vi "Remove signal offset - Intensity graph.vi"(8 "Y Scale.Offset and Multiplier":T2={"Offset"=-1.0, "Multiplier"=0.01}, 9 "X min & max":cluster{"X min":dbl, "X max":dbl}={"X min"=-0.4389, "X max"=0.4337}, 10 "Current offset to Subtract":T1, 11 "Data":dbl[][](graph)=array608x201[122208 elements]) -> (2 "element":dbl format="%#_6p", 3 "Data 2":dbl[][](graph))   [LabVIEW 2016]
uses:
  <vilib>/Utility/miscctls.llb/LVOffsetAndMultiplierTypeDef.ctl
panel:
  out "size(s)":i32[](array[numeric])=[608, 201]
  in  "Name":cluster{"X":string, "Y":string, "Z":string}={"X"="Vsd (V)", "Y"="VsgL (V)", "Z"="I (A)"}
  in  "Multiplier for Z":dbl=1.0
  out "Extracted offset signal":dbl[](graph)=[1.6161257772866977e-10, 1.6290791942826465e-10, 1.5574505344604935e-10, 1.336906684909418e-10, 1.3645714177751155e-10, 1.332223358181467e-10, 1.3050666232859227e-10, 1.2958403711911122e-10, 1.255087742878435e-10, 1.3438431801111367e-10, 1.3343613425025554e-10, 1.3796967145370057e-10, 1.3165183194433646e-10, 1.3668925850359432e-10, 1.3024287630588326e-10, 1.312700831203163e-10, 1.3321104247858227e-10, 1.3078678060118375e-10, 1.3530497739422364e-10, 1.3467471828812237e-10, 1.3723878465253679e-10, 1.3090930009882394e-10, 1.3122556497154024e-10, 1.3637331559158535e-10, 1.344618428788294e-10, 1.329384379410261e-10, 1.32436021964744e-10, 1.3267536092655857e-10, 1.3166939739249612e-10, 1.3315326666398787e-10, 1.3353313321086935e-10, 1.308474998524559e-10, 1.3430606449651886e-10, 1.3299895953833615e-10, 1.3379868824903194e-10, 1.3910099477931292e-10, 1.3013451141656342e-10, 1.3022082409430547e-10, 1.3957589625922564e-10, 1.353665592030564e-10, 1.3333443920084868e-10, 1.2848465625085147e-10, 1.3235016346451685e-10, 1.3493515356938516e-10, 1.3174423441498757e-10, 1.315524302167768e-10, 1.285457690751685e-10, 1.3328905759556557e-10, 1.3343261772296814e-10, 1.294368748288793e-10, 1.3434974891423252e-10, 1.2493174353418366e-10, 1.2818569417874195e-10, 1.375972145178948e-10, 1.3316519661996614e-10, 1.333160552162926e-10, 1.2807061594750737e-10, 1.2837747878228045e-10, 1.2925343445455244e-10, 1.3187529753832618e-10, 1.303560901885644e-10, 1.2711863941612015e-10, 1.2862070842066765e-10, 1.3111395651860157e-10, 1.2731619492783272e-10, 1.2928610264790122e-10, 1.3261741388716716e-10, 1.2936618128288814e-10, 1.3073484114123304e-10, 1.357022259458576e-10, 1.3308722303545194e-10, 1.2582991169744356e-10, 1.272984956323385e-10, 1.3313625085863706e-10, 1.3666798901102487e-10, 1.348284928206016e-10, 1.3155661735756067e-10, 1.2828337996704524e-10, 1.3817686001654687e-10, 1.313006770472531e-10, 1.3364094251474462e-10, 1.3219431956575055e-10, 1.2823138544113563e-10, 1.3058194682897394e-10, 1.2786306903663163e-10, 1.2121257776609541e-10, 1.2457836181502408e-10, 1.139019801741067e-10, -1.0289514736158215e-11, -1.079126256422265e-11, -7.17833194497521e-12, -1.1508360528901278e-11, -7.041294289787728e-12, -1.8425793356464854e-12, -7.342603760193337e-12, -1.182717940700916e-12, -9.257090530286378e-12, -1.1030122399284753e-11, 1.9500509432488837e-12, -2.0305343072338042e-12, 0.0, -6.0100382391542484e-12, -4.203032848042199e-12, -2.684888642627792e-12, -7.957273634973165e-13, 1.4131901363671778e-12, -6.5089009799810054e-12, -2.0573930093206007e-11, -2.0358993421467135e-11, -6.9621557217127364e-12, -2.375665809998132e-11, -3.8849048832914105e-11, -3.40603738443531e-11, -3.398990191858145e-11, -3.0637047451175085e-11, -2.2899999439023835e-11, -2.160057999761124e-11, -1.5155754435618327e-11, -1.6612365052405662e-11, -7.496874402767932e-12, 4.0679122982308985e-12, 3.484823081717634e-12, 7.539548185526302e-12, 2.2883162223965076e-11, 3.612015868987455e-11, 4.12107508832986e-11, 5.259279190531737e-11, 6.382994367033885e-11, 7.925386497350511e-11, 9.582310033816973e-11, 1.2233945274450482e-10, 1.3404805153739542e-10, 1.504789486211168e-10, 1.5513285360655564e-10, 1.5849933959225985e-10, 1.6380336707627032e-10, 1.5601485639021136e-10, 1.6243365043665102e-10, 1.6160236206965832e-10, 1.569039909026025e-10, 1.6402955480249391e-10, 1.589862609320719e-10, 1.5946189955419486e-10, 1.6003257363554858e-10, 1.6367793008706394e-10, 1.659416302854724e-10, 1.5812137434548563e-10, 1.5761297399206657e-10, 1.6304606686665208e-10, 1.6338092311678462e-10, 1.6211296267861397e-10, 1.6535008390287574e-10, 1.6378447086644309e-10, 1.626831696496228e-10, 1.6777616064733802e-10, 1.603554628703283e-10, 1.616490153232151e-10, 1.6545577071393482e-10, 1.6179943672467718e-10, 1.6279661934947987e-10, 1.613769684527713e-10, 1.583926399368027e-10, 1.6376811645845825e-10, 1.6323240508357437e-10, 1.6543880053438678e-10, 1.6528216102528657e-10, 1.6746161450290526e-10, 1.6677610756623038e-10, 1.6406096819225243e-10, 1.6722502777785532e-10, 1.6381689845148476e-10, 1.576670898084429e-10, 1.6132843232637722e-10, 1.6138399931044358e-10, 1.6438727958969843e-10, 1.6119104030445377e-10, 1.6104395522851581e-10, 1.605087961623316e-10, 1.6533483542777352e-10, 1.6368393333658942e-10, 1.6432402719593648e-10, 1.6050620752896467e-10, 1.6553026180986872e-10, 1.6406674934837046e-10, 1.6377560146908163e-10, 1.6471061202981615e-10, 1.5749289251977975e-10, 1.6352124520132882e-10, 1.5945542627026614e-10, 1.5776996738345193e-10, 1.625348331476063e-10, 1.6038408159454676e-10, 1.6593264339503264e-10, 1.6685034644763363e-10, 1.65278743352013e-10, 1.6218731478513443e-10, 1.5914953995849366e-10, 1.591945024726289e-10, 1.6051357090587566e-10, 1.6687615058269173e-10, 1.6067392288733536e-10]
  out "Array":dbl[][](array[numeric]) format="%#_6p"
  out "X Scale.Offset and Multiplier":T2={"Offset"=-0.4389, "Multiplier"=0.0014351973684210526}
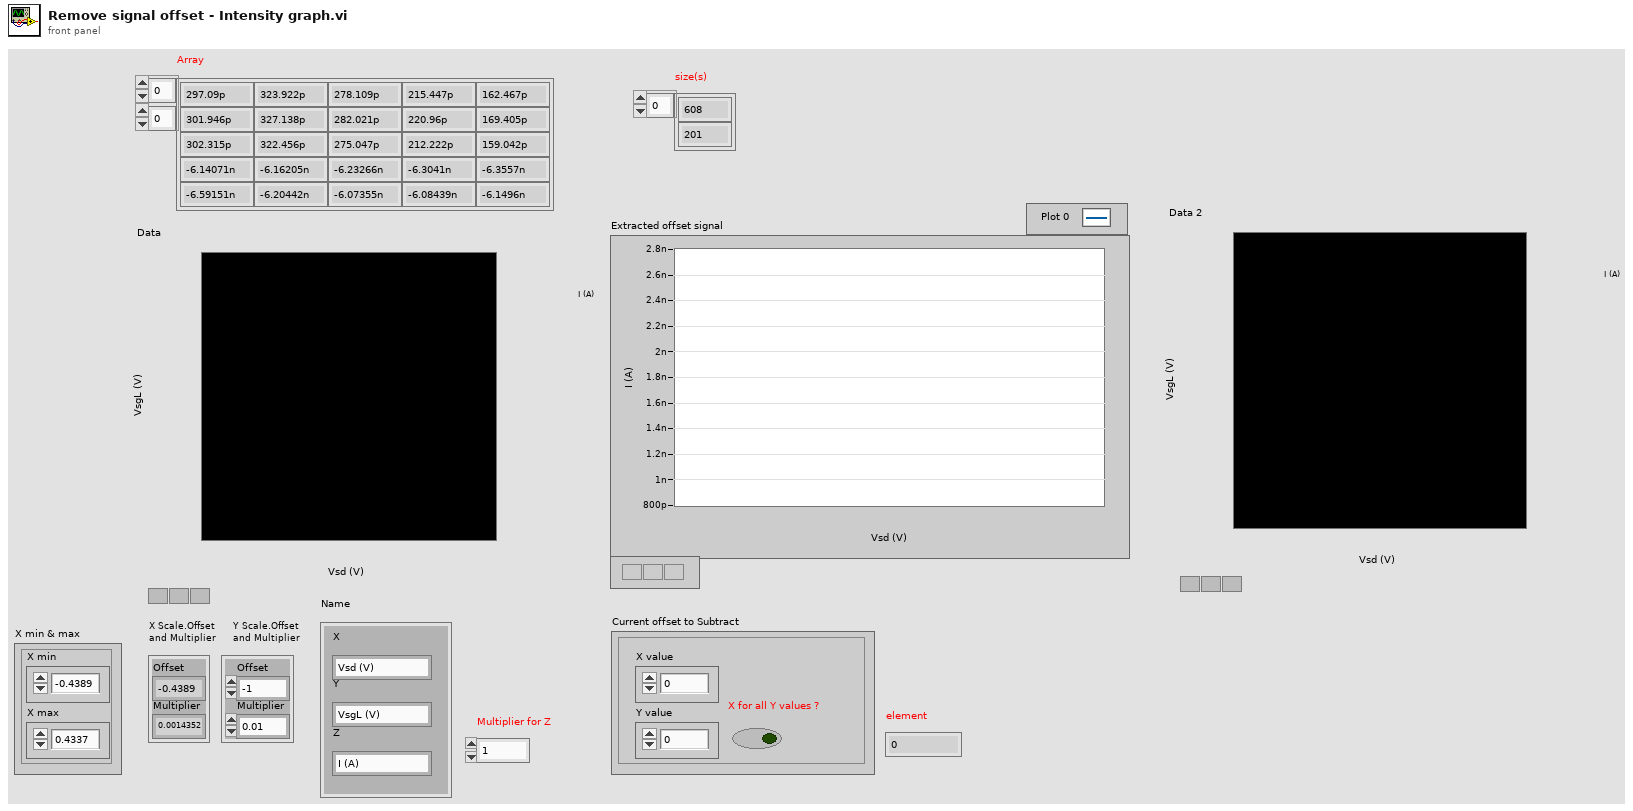
[diagram p1: front panel]
types:
  T1 = cluster{"X value":dbl, "Y value":dbl, "X for all Y values ?":bool}
  T2 = typedef "LVOffsetAndMultiplierTypeDef.ctl" = cluster{"Offset":dbl, "Multiplier":dbl}
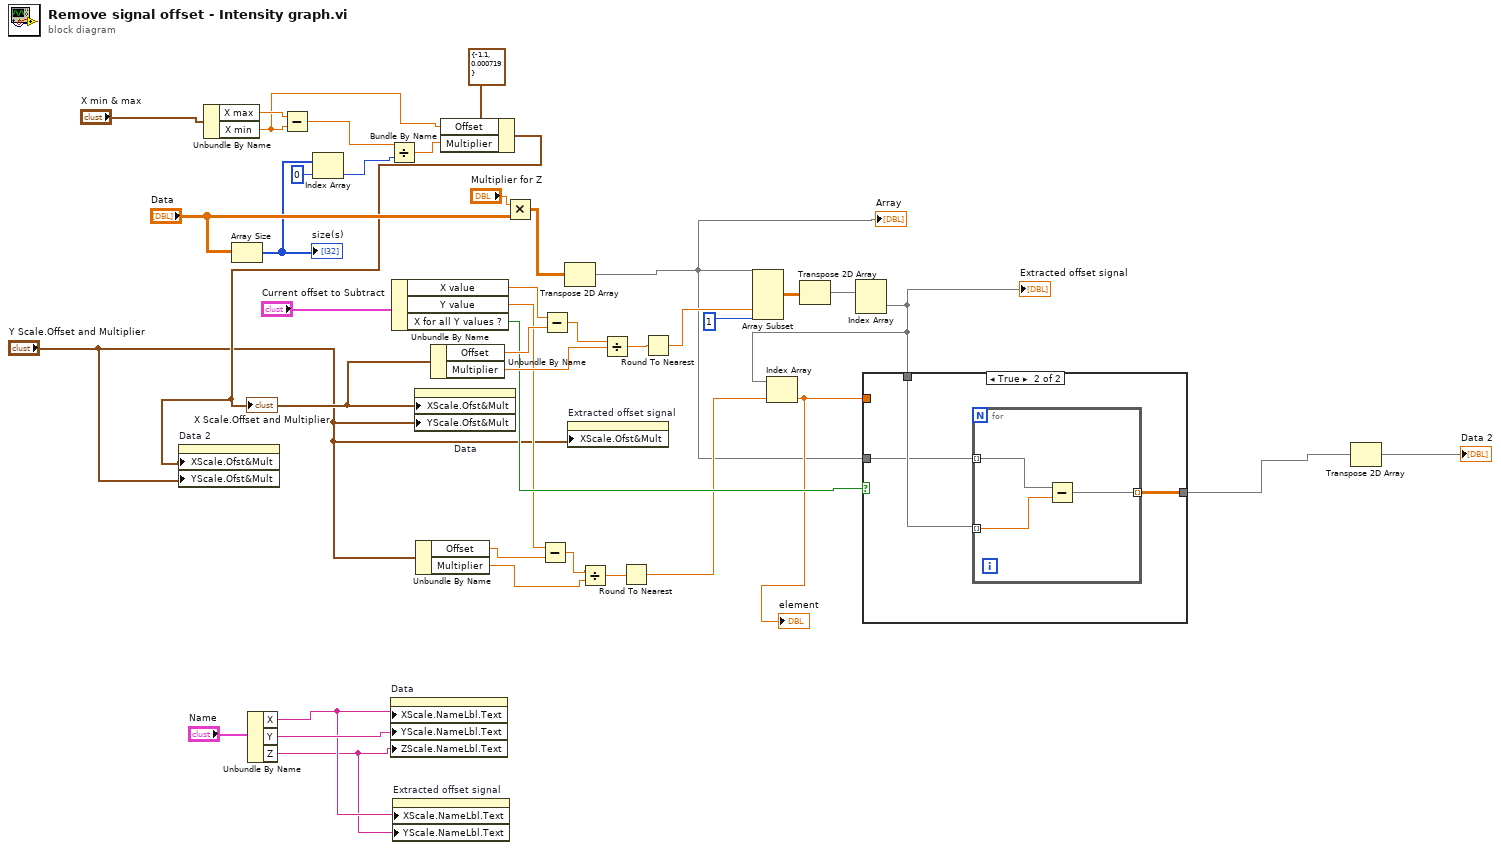
[diagram p0: block diagram]
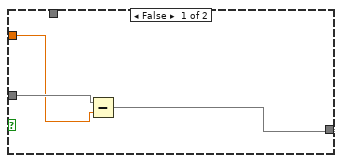
[diagram p2: hidden frame]
diagram:
  n1 = Unbundle By Name("X min & max") -> ("X max"=w8:dbl, "X min"=w4:dbl)
  n2 = Array Size(array="Data") -> (size(s)=w11:i32[])
  "size(s)" <- w11
  n3 = Unbundle By Name("Name") -> ("X"=w16:string, "Y"=w17:string, "Z"=w15:string)
  n4 = Subtract(x=w8, y=w4) -> (x-y=w6:dbl)
  n5 = Index Array(array=w11, index=0) -> (element=w7:i32)
  n6 = Divide(x=w6, y=w7) -> (x/y=w3:dbl)
  n7 = property on="Data" class="IntGraph (strict)"("XScale.NameLbl.Text"=w16, "YScale.NameLbl.Text"=w17, "ZScale.NameLbl.Text"=w15) -> ()  [unwired: 2 in, 2 out]
  n8 = Unbundle By Name("Current offset to Subtract") -> ("X value"=w39:dbl, "Y value"=w22:dbl, "X for all Y values ?"=w27:bool)
  n9 = property on="Extracted offset signal" class="WFGraph (strict)"("XScale.NameLbl.Text"=w16, "YScale.NameLbl.Text"=w15) -> ()  [unwired: 2 in, 2 out]
  n10 = Unbundle By Name("Y Scale.Offset and Multiplier") -> ("Offset"=w24:dbl, "Multiplier"=w23:dbl)
  n11 = Bundle By Name(cluster=T2 {"Offset"=-1.1, "Multiplier"=0.000719} ("X Scale.Offset and Multiplier"), "Offset"=w4, "Multiplier"=w3) -> (w2:T2)
  "X Scale.Offset and Multiplier" <- w2
  n12 = property on="Data 2" class="IntGraph (strict)"("XScale.Ofst&Mult"=w2, "YScale.Ofst&Mult"="Y Scale.Offset and Multiplier") -> ()  [unwired: 2 in, 2 out]
  n13 = property on="Data" class="IntGraph (strict)"("XScale.Ofst&Mult"=w2, "YScale.Ofst&Mult"="Y Scale.Offset and Multiplier") -> ()  [unwired: 2 in, 2 out]
  n14 = Unbundle By Name(w2) -> ("Offset"=w38:dbl, "Multiplier"=w36:dbl)
  n15 = Multiply(x="Multiplier for Z", y="Data") -> (x*y=w14:dbl[][])
  n16 = Subtract(x=w22, y=w24) -> (x-y=w21:dbl)
  n17 = Subtract(x=w39, y=w38) -> (x-y=w37:dbl)
  n18 = Transpose 2D Array(2D array=w14) -> (transposed array=w13:dbl[][])
  "Array" <- w13
  n19 = property on="Extracted offset signal" class="WFGraph (strict)"("XScale.Ofst&Mult"="Y Scale.Offset and Multiplier") -> ()  [unwired: 2 in, 2 out]
  n20 = Divide(x=w21, y=w23) -> (x/y=w20:dbl)
  n21 = Divide(x=w37, y=w36) -> (x/y=w35:dbl)
  n22 = Round To Nearest(number=w20) -> (nearest integer value=w19:dbl)
  n23 = Round To Nearest(number=w35) -> (nearest integer value=w32:dbl)
  n24 = Array Subset(array=w13, index (col)=w32, length (col)=1 ("length")) -> (w34:dbl[][])  [unwired: 2 in]
  n25 = Transpose 2D Array(2D array=w34) -> (transposed array=w30:dbl[][])
  n26 = Index Array(array=w30) -> (element=w26:dbl[])  [unwired: 2 in]
  "Extracted offset signal" <- w26
  n27 = Index Array(array=w26, index=w19) -> (element=w25:dbl)
  "element" <- w25
  n28 = case shown="True" w27 {
    tunnel: [w41 w46] -> w29
    tunnel: w26 -> [_ w45]
    tunnel: w13 -> [w43 w44]
    tunnel: w25 -> [w42 _]
    frame False {
      n29 = Subtract(x=w43, y=w42) -> (x-y=w41:dbl[][])
    }
    frame True {
      n30 = for {
        tunnel: w44 -> [w49] mode=indexing
        tunnel: w45 -> [w48] mode=indexing
        tunnel: [w47] -> w46 mode=indexing
        n31 = Subtract(x=w49, y=w48) -> (x-y=w47:dbl[])
      }
    }
  }
  n32 = Transpose 2D Array(2D array=w29) -> (transposed array=→"Data 2":dbl[][])
